vi "save_MPS_spectroscopy_hdf.vi"(0 "file path":path, 1 "Device Name":tag="DAQ2", 2 "Phase Rx over time":dbl[][](array[numeric]), 3 "Mag Rx over time":dbl[][](array[numeric]), 5 "TxRx_Params":T1={"sample rate"=1000000.0, "Tx freq"=23809.52380952381, "Tx amp"=1.5, "Tx cycles\nSpectroscopy"=500.0, "Bias amp"=2.0, "Bias freq"=11.904761904761905, "Receive range"=5.0, "Bias Periods\nMagnetometry"=5.0, "Tx Freq Division Factor"=42.0, "Drive Periods per Bias"=2000.0, "TX harmonics"=[52631.57894736842, 78947.36842105263, 105263.15789473684, 131578.94736842104, 157894.73684210525, 184210.52631578947, 210526.31578947368, 236842.1052631579]} {"TX harmonics" format="%#_6p"}, 7 "Rx_f0-f8 Units":string, 9 "Time Domain Cluster":T2={"Drive IMon"=array[500000 elements], "Rx Time Domain"=array[500000 elements], "Rx Empty Bore"=array[500000 elements], "BMon"=array[500000 elements], "Bias IMon"=array[500000 elements], "TF-Corr-MagOverTime"=[], "Interpolated Rx TF-Mag"=[], "Interpolated Rx TF-Phase"=[]}, 11 "Sample MetaData Cluster":T5={"Sample Volume (uL)"=5.0, "Sample Mass (ug)"=5.0, "Sample Conc(mg/mL)"=5.0, "Sample Temperature (C)"=5.0, "Batch Num"=5.0, "Batch Name"="", "Solute"="", "Solvent"="", "Sample Description"=""}, 12 "Study and Experiment Description":T4={"Study Number"=5, "Study Name"="", "UUID"="", "GUI Open Time"="", "Notes"=""}, 13 "Sample in_vs_Out":dbl[](array[numeric]), 14 "Scanner Description":T3={"Scanner Name"="", "Hardware description"="", "Preamplifier Used"="", "Preamp Gain"=5.0, "Drive Amplifier"="", "Bias Amplifier"="", "Drive Current Monitor"="", "Bias Current Monitor"=""}, 15 "Points from home to max":i32) -> ()   [LabVIEW 2021]
uses:
  <vilib>/UPVI/lvhdf5/file.llb/LVH5F Operation.ctl
  <vilib>/Utility/miscctls.llb/LVRectTypeDef.ctl
  <vilib>/UPVI/lvhdf5/group.llb/H5G_obj_t.ctl
  <vilib>/UPVI/lvhdf5/dataset.llb/LVH5D Operation.ctl
  <vilib>/UPVI/lvhdf5/attribute.llb/LVH5A Operation.ctl
  <vilib>/UPVI/lvhdf5/identifier.llb/Not an HDF5 Refnum Constant.vi
  <vilib>/UPVI/lvhdf5/attribute.llb/Write Multiple Attributes.vi
  MPS_global_variables.vi
  <vilib>/UPVI/lvhdf5/utility.llb/Select HDF5 Dialog.vi
  <vilib>/UPVI/lvhdf5/utility.llb/Select HDF5 Dialog (Object Only).vi
  <vilib>/UPVI/lvhdf5/dataset.llb/Simple H5Dwrite (Variant).vi
  <vilib>/UPVI/lvhdf5/common.llb/To HDF5 Ref.vi
  <vilib>/UPVI/lvhdf5/dataset.llb/H5Dclose.vi
  <vilib>/UPVI/lvhdf5/attribute.llb/LVH5 Write Attributes.xnode
  <vilib>/UPVI/lvhdf5/library.llb/HDF5 Ref.ctl
  <vilib>/UPVI/lvhdf5/dataset.llb/Simple H5Dwrite.xnode
  <vilib>/UPVI/lvhdf5/dataset.llb/Write Dataset with Attributes.xnode
  <vilib>/UPVI/lvhdf5/attribute.llb/Cluster to Attribute Array.xnode
  <vilib>/Utility/error.llb/Error Cluster From Error Code.vi
  <vilib>/UPVI/lvhdf5/dataset.llb/OpenCreateReplace Dataset by Element Type.vi
  <vilib>/UPVI/lvhdf5/dataspace.llb/H5Sselect_hyperslab.vi
  <vilib>/UPVI/lvhdf5/dataset.llb/H5Dwrite (Variant).vi
  <vilib>/UPVI/lvhdf5/dataset.llb/H5Dget_space.vi
  <vilib>/UPVI/lvhdf5/attribute.llb/private/LVH5AwriteWDTAttrs.vi
  <vilib>/UPVI/lvhdf5/dataspace.llb/H5Sclose.vi
  <vilib>/UPVI/lvhdf5/utility.llb/Select HDF5 Dialog (File and Object).vi
  <resource>/objmgr/daqmx.rc
  <vilib>/UPVI/lvhdf5/library.llb/HDF5 Ref.lvclass
  <vilib>/Utility/Data Type/Get Type Information.vi
  <vilib>/Utility/Data Type/NI_Data Type.lvlib
  <vilib>/Utility/Data Type/Get Cluster Information.vi
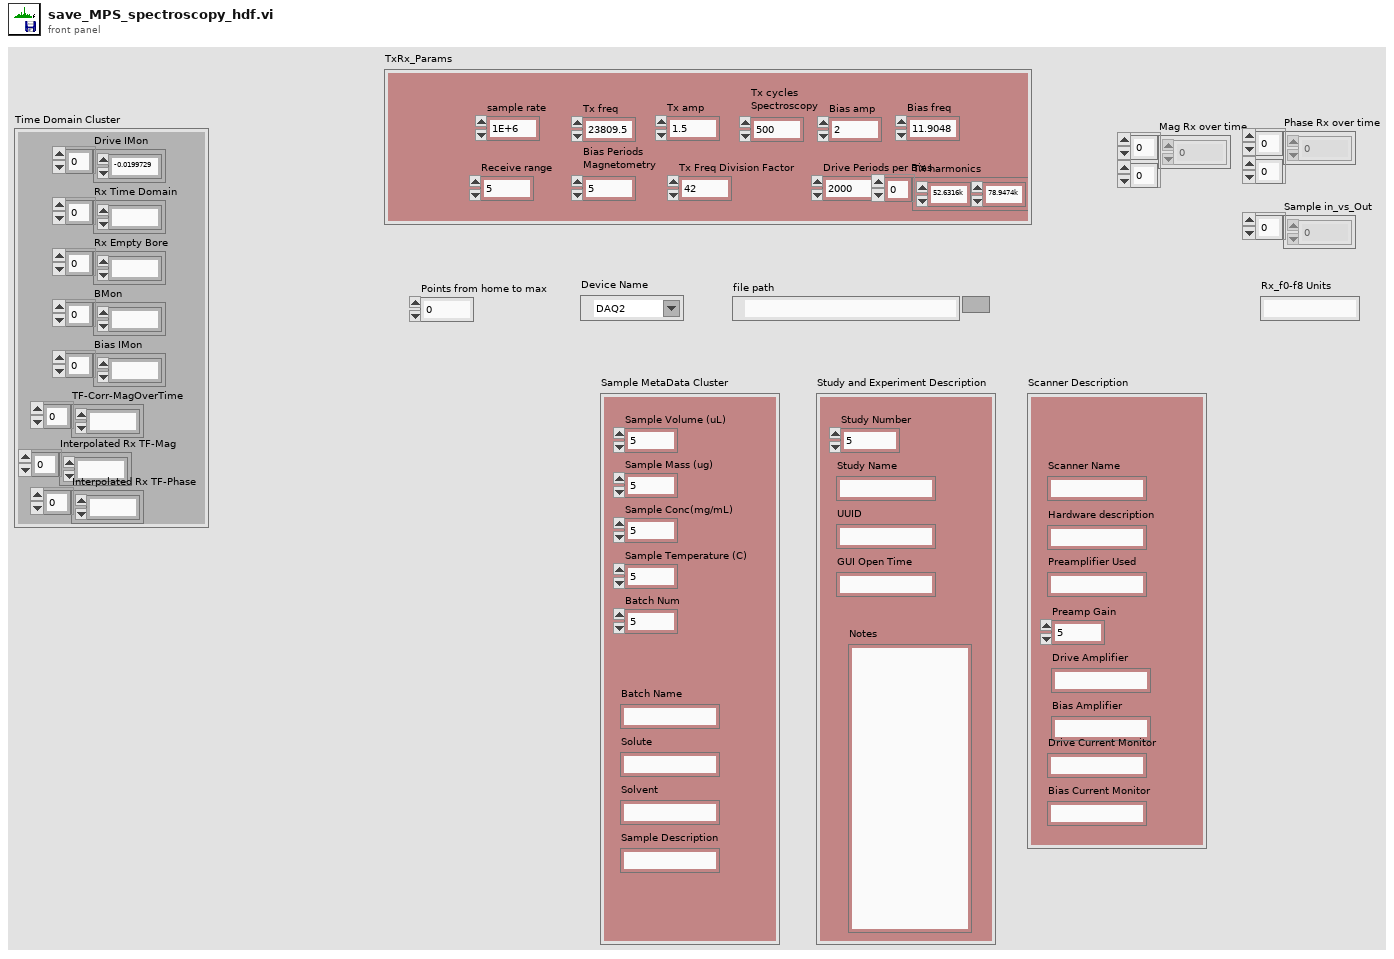
[diagram p1: front panel]
types:
  T1 = cluster{"sample rate":dbl, "Tx freq":dbl, "Tx amp":dbl, "Tx cycles\nSpectroscopy":dbl, "Bias amp":dbl, "Bias freq":dbl, "Receive range":dbl, "Bias Periods\nMagnetometry":dbl, "Tx Freq Division Factor":dbl, "Drive Periods per Bias":dbl, "TX harmonics":dbl[]}
  T2 = cluster{"Drive IMon":dbl[], "Rx Time Domain":dbl[], "Rx Empty Bore":dbl[], "BMon":dbl[], "Bias IMon":dbl[], "TF-Corr-MagOverTime":dbl[], "Interpolated Rx TF-Mag":dbl[], "Interpolated Rx TF-Phase":dbl[]}
  T3 = cluster{"Scanner Name":string, "Hardware description":string, "Preamplifier Used":string, "Preamp Gain":dbl, "Drive Amplifier":string, "Bias Amplifier":string, "Drive Current Monitor":string, "Bias Current Monitor":string}
  T4 = cluster{"Study Number":i64, "Study Name":string, "UUID":string, "GUI Open Time":string, "Notes":string}
  T5 = cluster{"Sample Volume (uL)":dbl, "Sample Mass (ug)":dbl, "Sample Conc(mg/mL)":dbl, "Sample Temperature (C)":dbl, "Batch Num":dbl, "Batch Name":string, "Solute":string, "Solvent":string, "Sample Description":string}
  T6 = typedef "LVH5F Operation.ctl" = enum16{"open", "open or create", "create or replace", "create or replace (with confirmation)", "create", "open (read only)"}
  T7 = typedef "HDF5 Ref.ctl" = refnum<class "HDF5 Ref.lvclass">
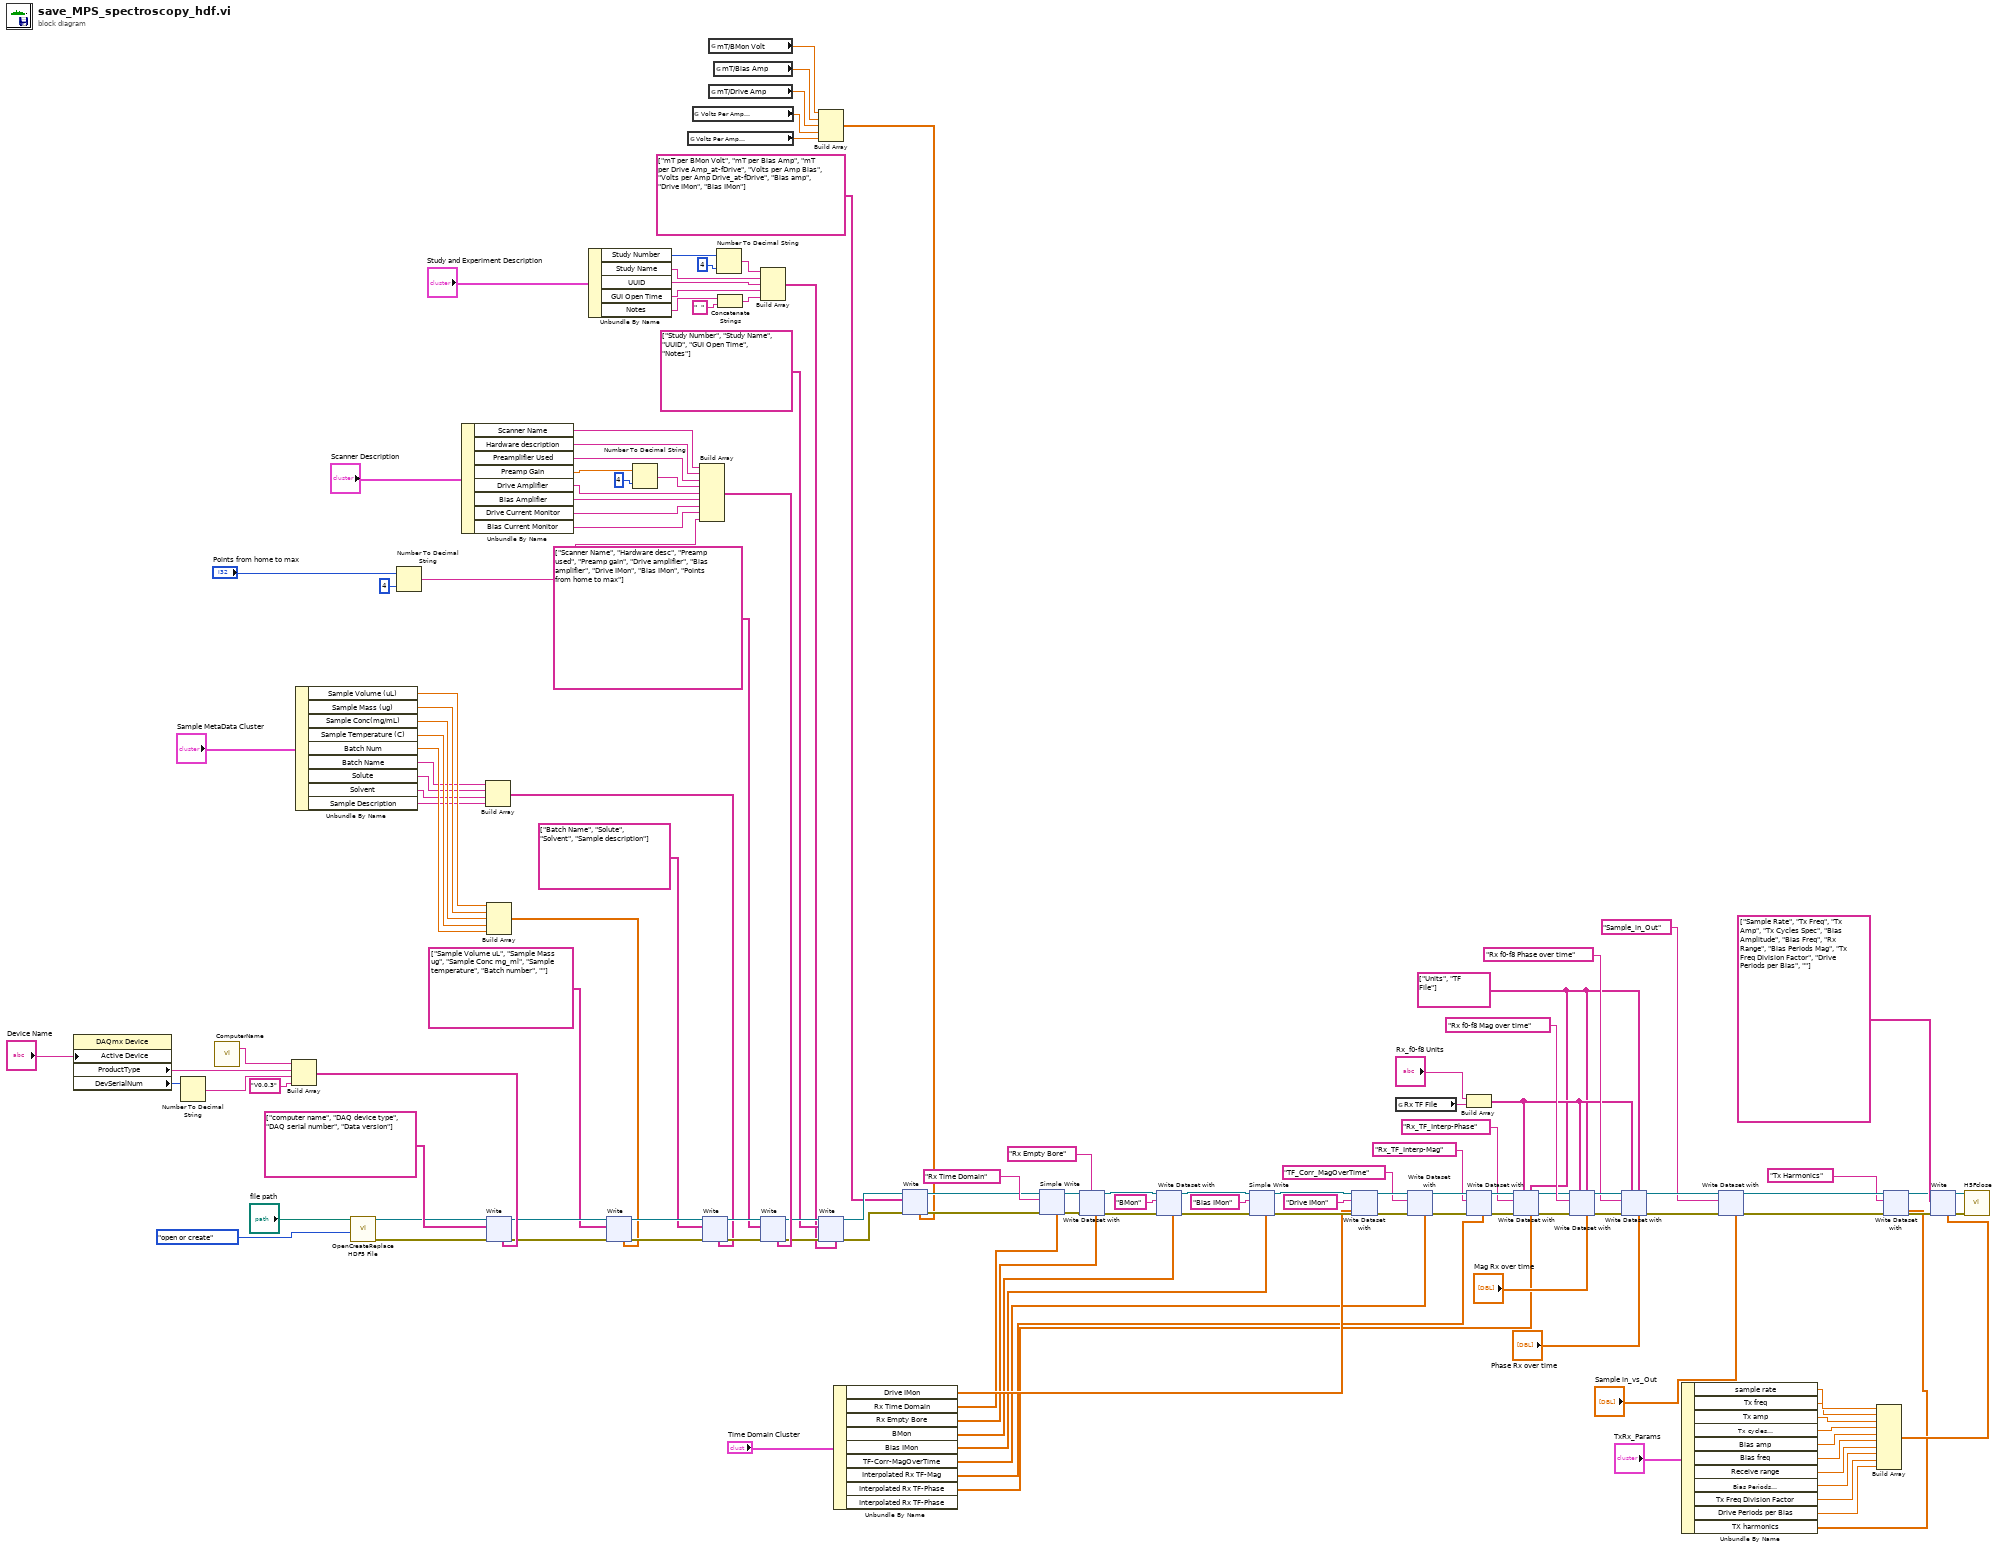
[diagram p0: block diagram]
diagram:
  w16 = string[] ["Units", "TF File"] ("Attribute Name(s)")
  n1 = property class="DAQmx Device"("Active Device"="Device Name") -> ("ProductType"=w134:string, "DevSerialNum"=w136:u32)  [unwired: 2 in, 2 out]
  n2 = Number To Decimal String(number=w136) -> (decimal integer string=w135:string)  [unwired: 1 in]
  n3 = call "ComputerName.vi"() -> ("String/Binary data"=w133:string)  [unwired: 4 in, 1 out]
  n4 = Build Array(w133, w134, w135, "V0.0.3" ("element")) -> (w132:string[])
  n5 = Unbundle By Name("Sample MetaData Cluster") -> ("Sample Volume (uL)"=w107:dbl, "Sample Mass (ug)"=w105:dbl, "Sample Conc(mg/mL)"=w104:dbl, "Sample Temperature (C)"=w103:dbl, "Batch Num"=w102:dbl, "Batch Name"=w101:string, "Solute"=w100:string, "Solvent"=w99:string, "Sample Description"=w98:string)
  n6 = call <vilib>:"OpenCreateReplace HDF5 File.vi"("function (open or create)"=LVH5F_Operation."open or create", "path"="file path") -> ("error out"=w127:errorcluster, "HDF5 Ref out"=w128:T7)  [unwired: 6 in]
  n7 = Number To Decimal String(number="Points from home to max", width (-)=i16 4) -> (decimal integer string=w2:string)
  n8 = Unbundle By Name("Scanner Description") -> ("Scanner Name"=w95:string, "Hardware description"=w94:string, "Preamplifier Used"=w93:string, "Preamp Gain"=w97:dbl, "Drive Amplifier"=w91:string, "Bias Amplifier"=w90:string, "Drive Current Monitor"=w89:string, "Bias Current Monitor"=w88:string)
  n9 = Build Array(w101, w100, w99, w98) -> (w79:string[])
  n10 = Build Array(w107, w105, w104, w103, w102) -> (w80:dbl[])
  n11 = xnode "Write"("HDF5 Ref"=w128, "error in (no error)"=w127, "Name(s)"=string[] ["computer name", "DAQ device type", "DAQ serial number", "Data version"], "Value(s)"=w132) -> ("HDF5 Ref out"=w126:T7, "error out"=w125:errorcluster)  [unwired: 1 in]
  n12 = Unbundle By Name("Study and Experiment Description") -> ("Study Number"=w86:i64, "Study Name"=w83:string, "UUID"=w82:string, "GUI Open Time"=w81:string, "Notes"=w33:string)
  n13 = xnode "Write"("HDF5 Ref"=w126, "error in (no error)"=w125, "Name(s)"=string[] ["Sample Volume uL", "Sample Mass ug", "Sample Conc mg_ml", "Sample temperature", "Batch number", ""], "Value(s)"=w80) -> ("HDF5 Ref out"=w114:T7, "error out"=w112:errorcluster)  [unwired: 1 in]
  n14 = Number To Decimal String(number=w97, width (-)=i16 4) -> (decimal integer string=w92:string)
  n15 = global read "MPS_global_variables.vi" "Volts Per Amp\nDrive"() -> (w7:dbl)
  n16 = global read "MPS_global_variables.vi" "Volts Per Amp\nBias"() -> (w8:dbl)
  n17 = Build Array(w95, w94, w93, w92, w91, w90, w89, w88, w2) -> (w78:string[])
  n18 = xnode "Write"("HDF5 Ref"=w114, "error in (no error)"=w112, "Name(s)"=string[] ["Batch Name", "Solute", "Solvent", "Sample description"], "Value(s)"=w79) -> ("HDF5 Ref out"=w113:T7, "error out"=w111:errorcluster)  [unwired: 1 in]
  n19 = global read "MPS_global_variables.vi" "mT/BMon Volt"() -> (w11:dbl)
  n20 = global read "MPS_global_variables.vi" "mT/Drive Amp"() -> (w9:dbl)
  n21 = global read "MPS_global_variables.vi" "mT/Bias Amp"() -> (w10:dbl)
  n22 = Number To Decimal String(number=w86, width (-)=i16 4) -> (decimal integer string=w84:string)
  n23 = Concatenate Strings(w33, "  " ("string")) -> (w32:string)
  n24 = Build Array(w84, w83, w82, w81, w32) -> (w74:string[])
  n25 = xnode "Write"("HDF5 Ref"=w113, "error in (no error)"=w111, "Name(s)"=string[] ["Scanner Name", "Hardware desc", "Preamp used", "Preamp gain", "Drive amplifier", "Bias amplifier", "Drive IMon", "Bias IMon", "Points from home to max"], "Value(s)"=w78) -> ("HDF5 Ref out"=w77:T7, "error out"=w76:errorcluster)  [unwired: 1 in]
  n26 = Build Array(w11, w10, w9, w8, w7) -> (w5:dbl[])
  n27 = xnode "Write"("HDF5 Ref"=w77, "error in (no error)"=w76, "Name(s)"=string[] ["Study Number", "Study Name", "UUID", "GUI Open Time", "Notes"], "Value(s)"=w74) -> ("HDF5 Ref out"=w15:T7, "error out"=w13:errorcluster)  [unwired: 1 in]
  n28 = Unbundle By Name("Time Domain Cluster") -> ("Drive IMon"=w72:dbl[], "Rx Time Domain"=w71:dbl[], "Rx Empty Bore"=w70:dbl[], "BMon"=w69:dbl[], "Bias IMon"=w68:dbl[], "TF-Corr-MagOverTime"=w34:dbl[], "Interpolated Rx TF-Mag"=w35:dbl[], "Interpolated Rx TF-Phase"=w19:dbl[])  [unwired: 1 out]
  n29 = xnode "Write"("HDF5 Ref"=w15, "error in (no error)"=w13, "Name(s)"=string[] ["mT per BMon Volt", "mT per Bias Amp", "mT per Drive Amp_at-fDrive", "Volts per Amp Bias", "Volts per Amp Drive_at-fDrive", "Bias amp", "Drive IMon", "Bias IMon"], "Value(s)"=w5) -> ("HDF5 Ref out"=w14:T7, "error out"=w12:errorcluster)  [unwired: 1 in]
  n30 = xnode "Simple Write"("Dataset Path"="Rx Time Domain", "error in (no error)"=w12, "HDF5 Path or Ref"=w14, "Data"=w71) -> ("HDF5 Ref out"=w138:T7, "error out"=w139:errorcluster)  [unwired: 4 in, 1 out]
  n31 = xnode "Write Dataset with"("Dataset Path"="Rx Empty Bore", "error in (no error)"=w139, "HDF5 Path or Ref"=w138, "Data"=w70) -> ("HDF5 Ref out"=w123:T7, "error out"=w122:errorcluster)  [unwired: 4 in, 1 out]
  n32 = xnode "Write Dataset with"("Dataset Path"="BMon", "error in (no error)"=w122, "HDF5 Path or Ref"=w123, "Data"=w69) -> ("HDF5 Ref out"=w120:T7, "error out"=w118:errorcluster)  [unwired: 4 in, 1 out]
  n33 = xnode "Simple Write"("Dataset Path"="Bias IMon", "error in (no error)"=w118, "HDF5 Path or Ref"=w120, "Data"=w68) -> ("HDF5 Ref out"=w119:T7, "error out"=w117:errorcluster)  [unwired: 4 in, 1 out]
  n34 = xnode "Write Dataset with"("Dataset Path"="Drive IMon", "error in (no error)"=w117, "HDF5 Path or Ref"=w119, "Data"=w72) -> ("HDF5 Ref out"=w38:T7, "error out"=w40:errorcluster)  [unwired: 4 in, 1 out]
  n35 = global read "MPS_global_variables.vi" "Rx TF File"() -> (w4:string)
  n36 = xnode "Write Dataset with"("Dataset Path"="TF_Corr_MagOverTime", "error in (no error)"=w40, "HDF5 Path or Ref"=w38, "Data"=w34) -> ("HDF5 Ref out"=w39:T7, "error out"=w41:errorcluster)  [unwired: 4 in, 1 out]
  n37 = Build Array("Rx_f0-f8 Units", w4) -> (w17:string[])
  n38 = xnode "Write Dataset with"("Dataset Path"="Rx_TF_Interp-Mag", "error in (no error)"=w41, "HDF5 Path or Ref"=w39, "Data"=w35) -> ("HDF5 Ref out"=w24:T7, "error out"=w22:errorcluster)  [unwired: 4 in, 1 out]
  n39 = xnode "Write Dataset with"("Dataset Path"="Rx_TF_Interp-Phase", "error in (no error)"=w22, "HDF5 Path or Ref"=w24, "Attribute Name(s)"=w16, "Attribute Value(s)"=w17, "Data"=w19) -> ("HDF5 Ref out"=w23:T7, "error out"=w21:errorcluster)  [unwired: 2 in, 1 out]
  n40 = xnode "Write Dataset with"("Dataset Path"="Rx f0-f8 Mag over time", "error in (no error)"=w21, "HDF5 Path or Ref"=w23, "Attribute Name(s)"=w16, "Attribute Value(s)"=w17, "Data"="Mag Rx over time") -> ("HDF5 Ref out"=w50:T7, "error out"=w49:errorcluster)  [unwired: 2 in, 1 out]
  n41 = xnode "Write Dataset with"("Dataset Path"="Rx f0-f8 Phase over time", "error in (no error)"=w49, "HDF5 Path or Ref"=w50, "Attribute Name(s)"=w16, "Attribute Value(s)"=w17, "Data"="Phase Rx over time") -> ("HDF5 Ref out"=w46:T7, "error out"=w45:errorcluster)  [unwired: 2 in, 1 out]
  n42 = Unbundle By Name("TxRx_Params") -> ("sample rate"=w65:dbl, "Tx freq"=w64:dbl, "Tx amp"=w63:dbl, "Tx cycles\nSpectroscopy"=w62:dbl, "Bias amp"=w61:dbl, "Bias freq"=w60:dbl, "Receive range"=w59:dbl, "Bias Periods\nMagnetometry"=w58:dbl, "Tx Freq Division Factor"=w52:dbl, "Drive Periods per Bias"=w53:dbl, "TX harmonics"=w25:dbl[])
  n43 = xnode "Write Dataset with"("Dataset Path"="Sample_in_Out", "error in (no error)"=w45, "HDF5 Path or Ref"=w46, "Data"="Sample in_vs_Out") -> ("HDF5 Ref out"=w30:T7, "error out"=w29:errorcluster)  [unwired: 4 in, 1 out]
  n44 = Build Array(w65, w64, w63, w62, w61, w60, w59, w58, w52, w53) -> (w51:dbl[])
  n45 = xnode "Write Dataset with"("Dataset Path"="Tx Harmonics", "error in (no error)"=w29, "HDF5 Path or Ref"=w30, "Data"=w25) -> ("HDF5 Ref out"=w27:T7, "error out"=w28:errorcluster)  [unwired: 4 in, 1 out]
  n46 = xnode "Write"("HDF5 Ref"=w27, "error in (no error)"=w28, "Name(s)"=string[] ["Sample Rate", "Tx Freq", "Tx Amp", "Tx Cycles Spec", "Bias Amplitude", "Bias Freq", "Rx Range", "Bias Periods Mag", "Tx Freq Division Factor", "Drive Periods per Bias", ""], "Value(s)"=w51) -> ("HDF5 Ref out"=w67:T7, "error out"=w57:errorcluster)  [unwired: 1 in]
  n47 = call <vilib>:"H5Fclose.vi"("error in (no error)"=w57, "HDF5 Ref"=w67) -> ()  [unwired: 7 in, 1 out]
